vi "Tester - Chirp_FPGA_prototype.vi"() -> ()   [LabVIEW 2015]
panel:
  out "ChirpData accepted":csg[](array[numeric])
  out "Re Chirp Out Sorted":sgl[](array[numeric])
  out "Im Chirp Out Sorted":sgl[](array[numeric])
  out "Re Chirp Out":sgl[](array[numeric])
  out "Im Chirp Out":sgl[](array[numeric])
  out "Im Error":sgl[](array[numeric])
  out "Re Error":sgl[](array[numeric])
  out "Current Iteration":i32=262143
  out "% Error":sgl[](array[numeric]) format="%_8g"
  in  "Chirp/Fft Pair 1 - Chirp Rate":dbl=0.00554556
  in  "ChirpData":csg[](array[numeric])=array[262144 elements] format="%_8g"
  # "262144"
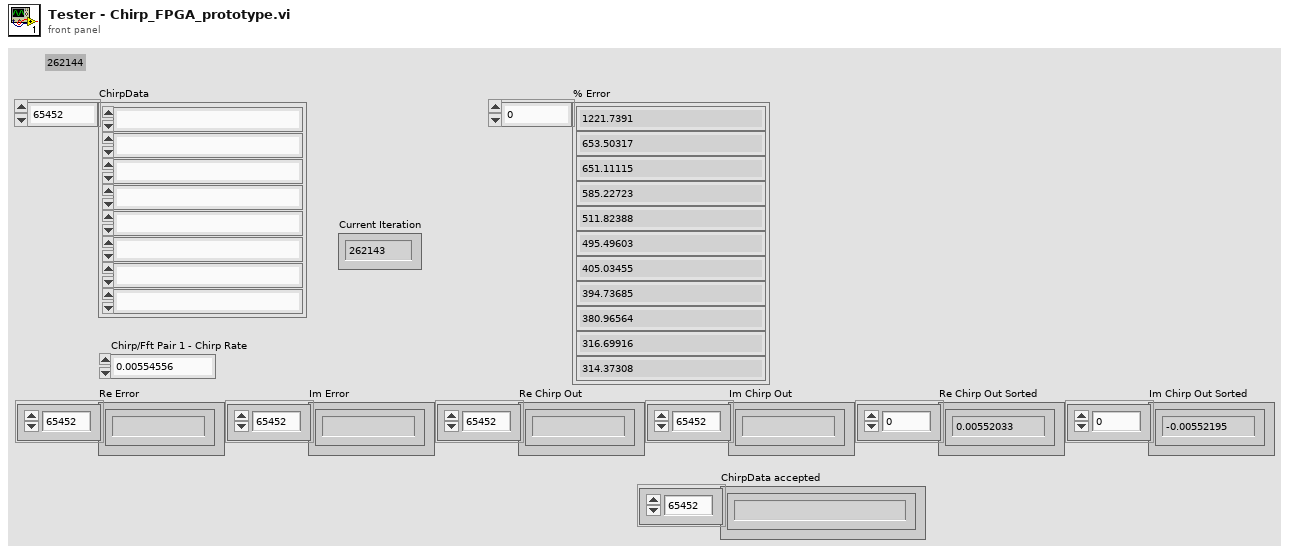
[diagram p1: front panel]
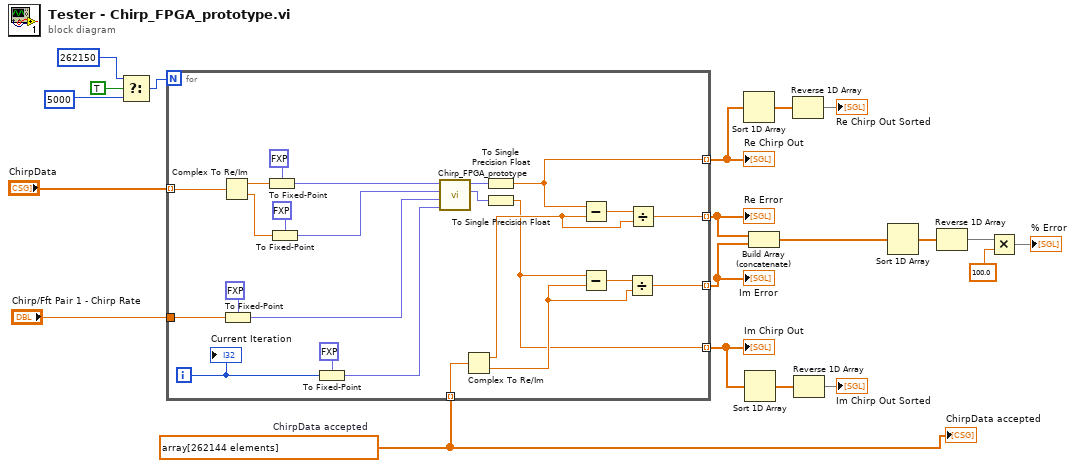
[diagram p0: block diagram]
diagram:
  w1 = csg[] array[262144 elements]  # ChirpData accepted
  n1 = Select(t=262150, s=TRUE, f=5000) -> (s? t:f=w4:i32)
  n2 = for {
    N: w4 -> [_]
    tunnel: "Chirp/Fft Pair 1 - Chirp Rate" -> [w37]
    tunnel: "ChirpData" -> [w44] mode=indexing
    tunnel: w1 -> [w29] mode=indexing
    tunnel: [w26] -> w17 mode=indexing
    tunnel: [w24] -> w11 mode=indexing
    tunnel: [w22] -> w8 mode=indexing
    tunnel: [w21] -> w7 mode=indexing
    i -> [w36]
    n3 = Complex To Re/Im(x + iy=w44) -> (x=w43:sgl, y=w39:sgl)
    n4 = To Fixed-Point(fixed-point type=fxp<+/-,64,2> 0.0 ("Chirp/Fft Pair 1 - Chirp Rate"), number=w37) -> (fixed-point=w32:fxp<+/-,64,2>)
    n5 = To Fixed-Point(fixed-point type=fxp<+/-,64,2> 0.0 ("Real In"), number=w43) -> (fixed-point=w42:fxp<+/-,64,2>)
    n6 = To Fixed-Point(fixed-point type=fxp<+/-,64,2> 0.0 ("Imaginary In"), number=w39) -> (fixed-point=w38:fxp<+/-,64,2>)
    n7 = To Fixed-Point(fixed-point type=fxp<+/-,64,32> 0.0 ("Iteration"), number=w36) -> (fixed-point=w35:fxp<+/-,64,32>)
    n8 = call "Chirp_FPGA_prototype.vi"("Iteration"=w35, "Chirp/Fft Pair 1 - Chirp Rate"=w32, "Imaginary In"=w38, "Real In"=w42) -> ("Imaginary Out"=w30:fxp<+/-,64,2>, "Real Out"=w31:fxp<+/-,64,2>)  [unwired: 6 in]
    n9 = Complex To Re/Im(x + iy=w29) -> (x=w25:sgl, y=w23:sgl)
    n10 = To Single Precision Float(number=w31) -> (single precision float=w22:sgl)
    n11 = To Single Precision Float(number=w30) -> (single precision float=w21:sgl)
    n12 = Subtract(x=w22, y=w25) -> (x-y=w28:sgl)
    n13 = Subtract(x=w21, y=w23) -> (x-y=w27:sgl)
    n14 = Divide(x=w27, y=w23) -> (x/y=w24:sgl)
    n15 = Divide(x=w28, y=w25) -> (x/y=w26:sgl)
    "Current Iteration" <- w36
  }
  "Re Error" <- w17
  "Im Error" <- w11
  "Im Chirp Out" <- w7
  "Re Chirp Out" <- w8
  n16 = Sort 1D Array(array=w8) -> (sorted array=w10:sgl[])
  n17 = Sort 1D Array(array=w7) -> (sorted array=w9:sgl[])
  n18 = Build Array (concatenate)(w17, w11) -> (w16:sgl[])
  n19 = Reverse 1D Array(array=w10) -> (reversed array=→"Re Chirp Out Sorted":sgl[])
  n20 = Reverse 1D Array(array=w9) -> (reversed array=→"Im Chirp Out Sorted":sgl[])
  n21 = Sort 1D Array(array=w16) -> (sorted array=w15:sgl[])
  n22 = Reverse 1D Array(array=w15) -> (reversed array=w14:sgl[])
  n23 = Multiply(x=w14, y=sgl 100.0) -> (x*y=→"% Error":sgl[])
  "ChirpData accepted" <- w1
